vi "viewerDisplay.vi"(8 "error in (no error)":errorcluster, 9 "closeEvent":refnum<user-event>, 10 "snapperEvents":T1, 11 "Views.lvlib:Camera.lvlib:Snapper in":refnum<class "Snapper.lvclass">) -> (0 "error out":errorcluster, 3 "Views.lvlib:Camera.lvlib:Snapper out":refnum<class "Snapper.lvclass">)   [LabVIEW 2009]
uses:
  Snapper.lvclass
panel:
  out "y profile":cluster{"Pixels Line":sgl[], i32[]}(graph)
  out "X Profile":cluster{"x0":sgl, "dx":sgl, "Pixels Line":sgl[]}(graph)
  in  "Scrollbar":i32(c297)
  out "Path":path
  out "Image":T2(plugin-control)
  in  "close":bool
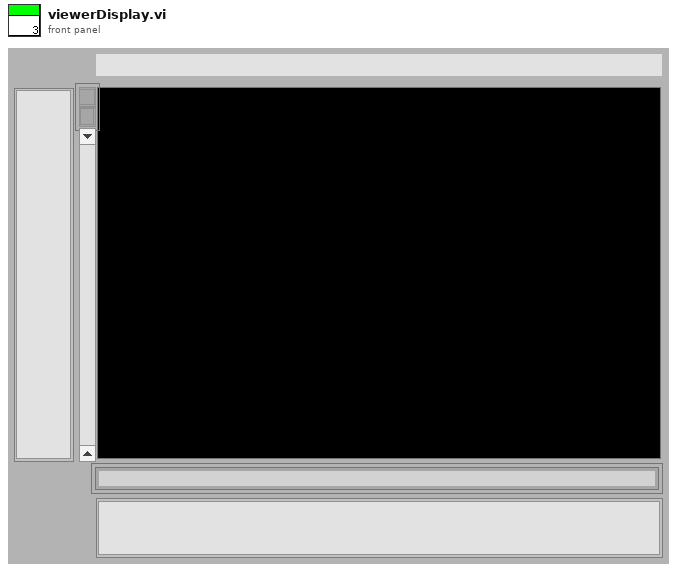
[diagram p1: front panel]
types:
  T1 = cluster{"frontEndEvents":cluster{"snapShotEvent":refnum<user-event>, "stopShooting":refnum<user-event>, "userSnapShot":refnum<user-event>}, "backEndEvents":cluster{"picture":refnum<user-event>}}
  T2 = typedef "IMAQ Image.ctl" = refnum<image>
  T3 = cluster{"snapShotEvent":refnum<user-event>, "stopShooting":refnum<user-event>, "userSnapShot":refnum<user-event>}
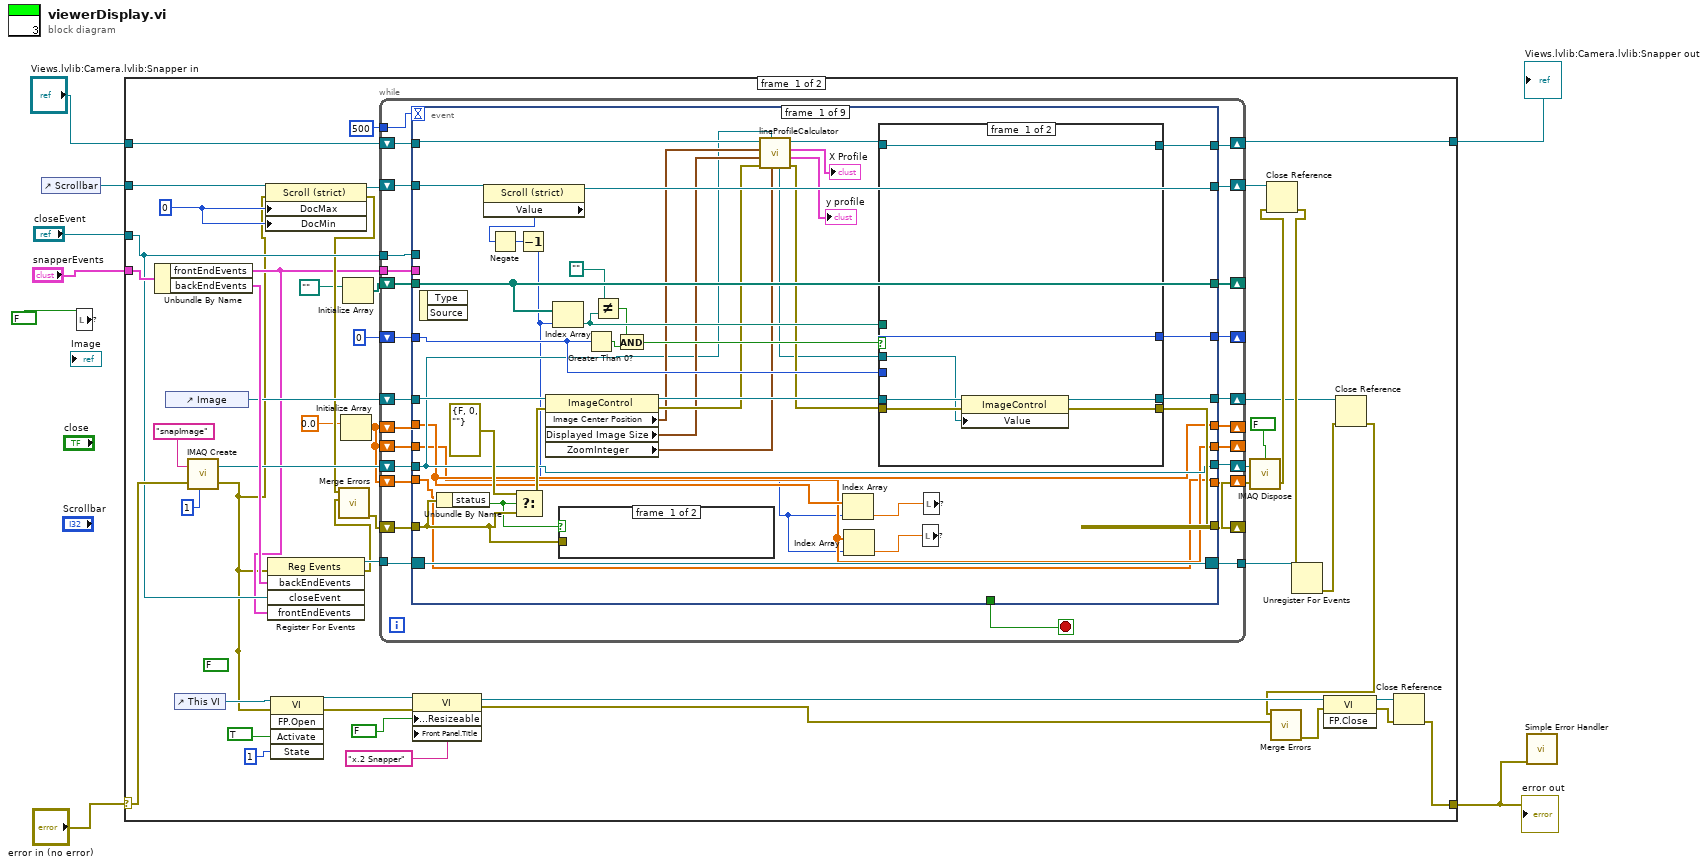
[diagram p0: block diagram]
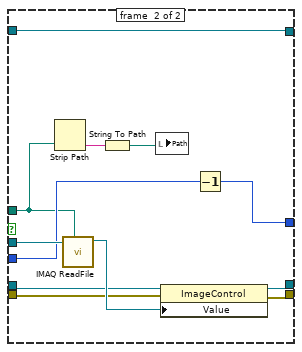
[diagram p2: hidden frame]
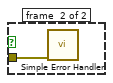
[diagram p3: hidden frame]
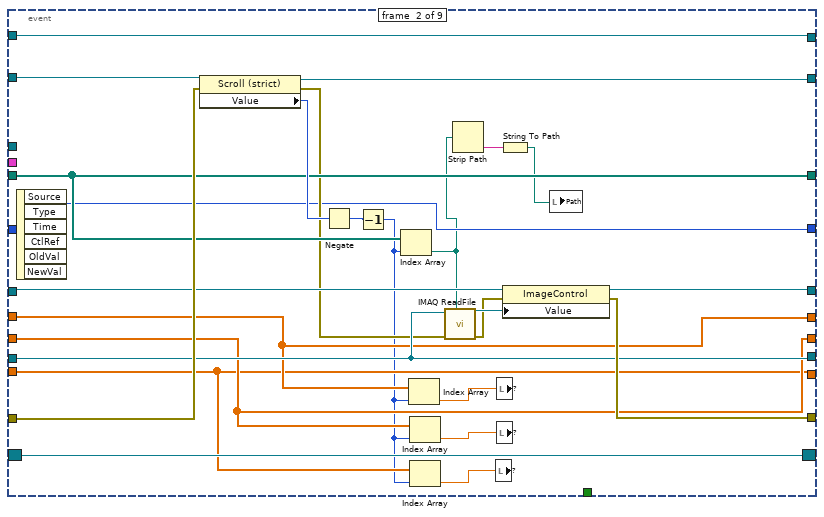
[diagram p4: hidden frame]
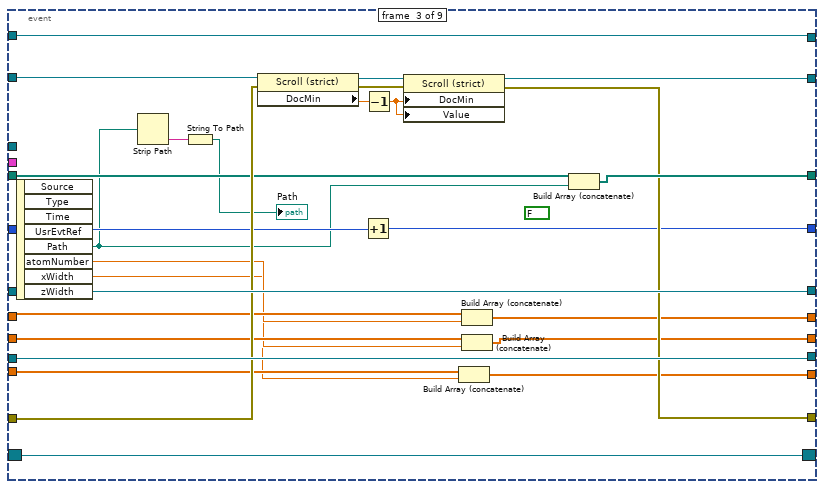
[diagram p5: hidden frame]
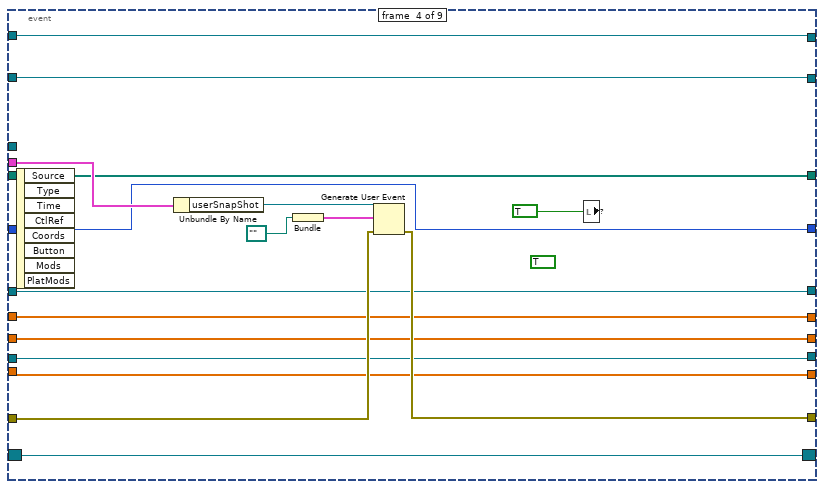
[diagram p6: hidden frame]
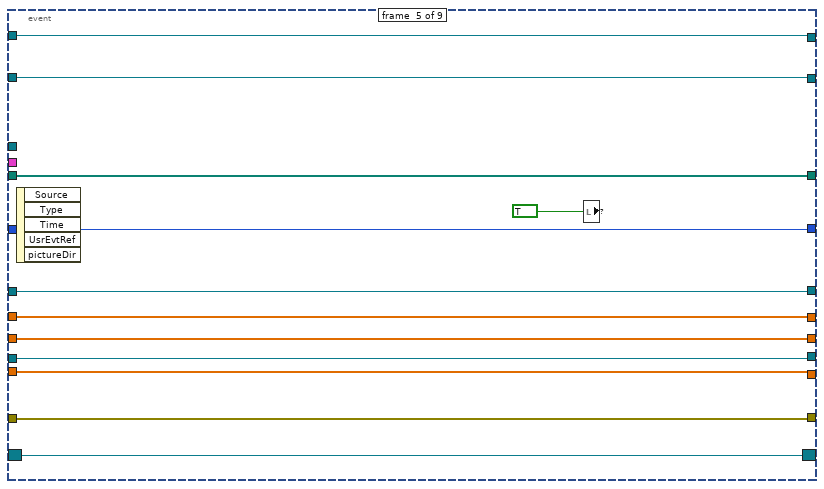
[diagram p7: hidden frame]
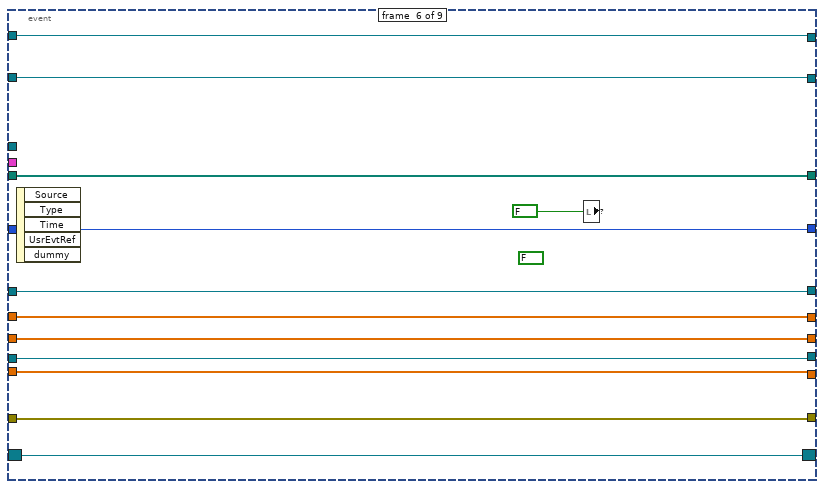
[diagram p8: hidden frame]
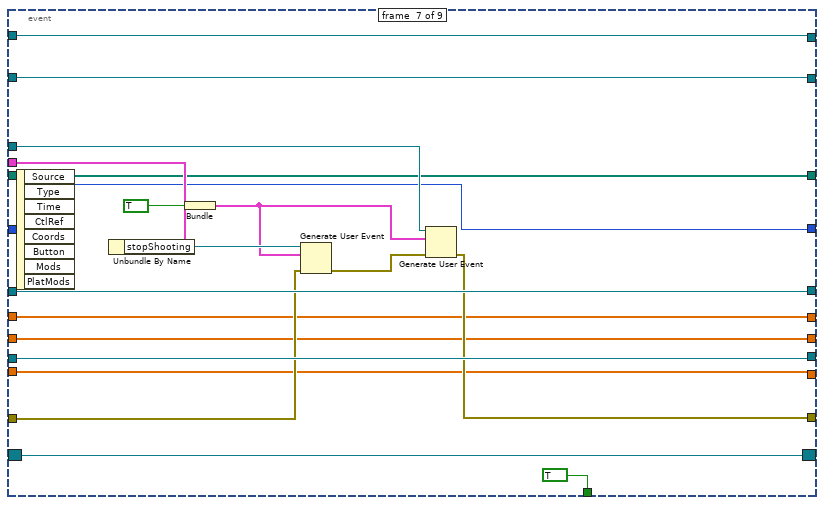
[diagram p9: hidden frame]
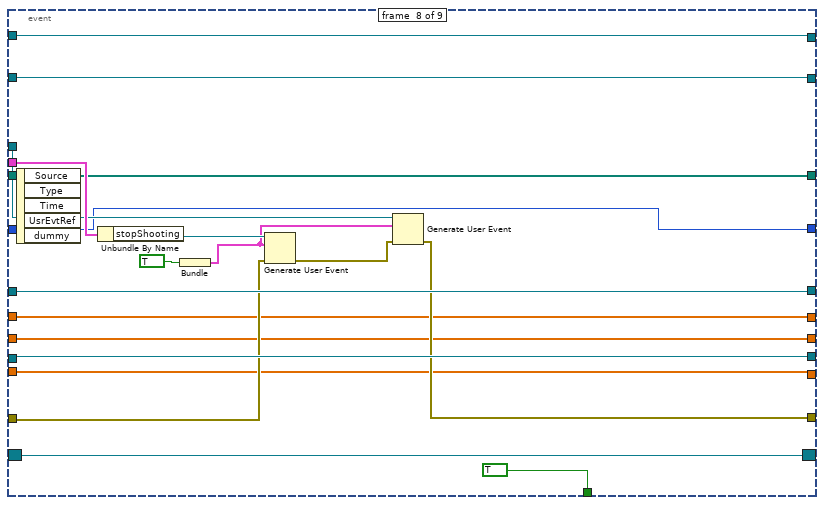
[diagram p10: hidden frame]
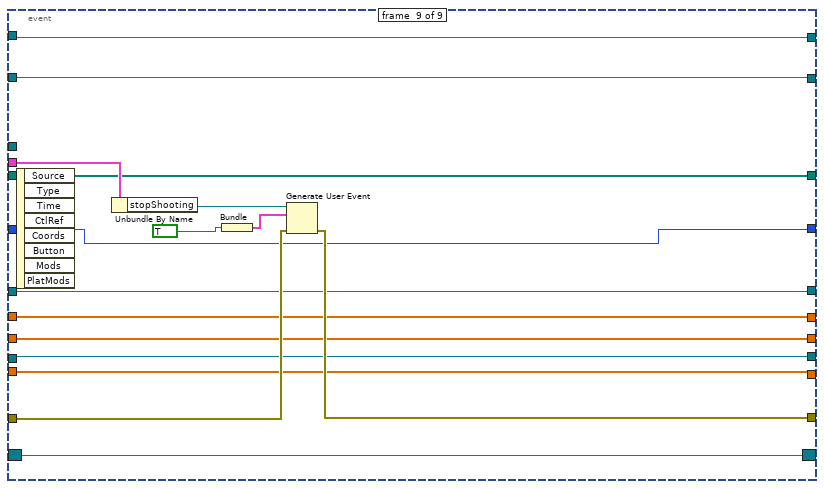
[diagram p11: hidden frame]
diagram:
  n1 = control-ref of="Scrollbar"() -> (w2:refnum<vi>)
  n2 = local write item#-1(FALSE) -> ()
  n3 = case shown="No Error" "error in (no error)" {
    selector: "error in (no error)" -> [w51 w296]
    tunnel: [w38 w296] -> w1
    tunnel: [w25 w295] -> w6
    tunnel: "Views.lvlib:Camera.lvlib:Snapper in" -> [w26 w295]
    tunnel: "snapperEvents" -> [w57 _]
    tunnel: "closeEvent" -> [w37 _]
    tunnel: w2 -> [w36 _]
    frame #0 {
      w18 = FALSE
      w34 = 0
      n4 = Unbundle By Name(w57) -> ("frontEndEvents"=w20:T3, "backEndEvents"=w55:cluster{"picture":refnum<user-event>})
      n5 = control-ref of="Image"() -> (w50:refnum<vi>)
      n6 = control-ref of="This VI"() -> (w44:refnum<vi>)
      n7 = call "IMAQ Create"("Image Name"="snapImage", "Image Type"=1, "error in (no error)"=w51) -> ("New Image"=w53:T2, "error out"=w19:errorcluster)  [unwired: 2 in]
      n8 = property class="Scroll (strict)"(reference=w36, error in=w19, "DocMax"=w34, "DocMin"=w34) -> (reference out=w35:refnum<vi>, error out=w33:errorcluster)
      n9 = register-events(error in=w19, w55, w37, w20) -> (reference out=w56:refnum<event-registration>, error out=w32:errorcluster)  [unwired: 1 in]
      n10 = invoke class="VI" method="FP.Open"(reference=w44, error in=w19, "Activate"=TRUE, "State"=1) -> (reference out=w40:refnum<vi>, error out=w39:errorcluster)  [unwired: 1 in, 3 out]
      n11 = call <vilib>:"Merge Errors.vi"("error in 2 (no error)"=w32, "error in 1 (no error)"=w33) -> ("error out"=w31:errorcluster)  [unwired: 5 in]
      n12 = Initialize Array(0.0) -> (w9:dbl[])  [unwired: 1 in]
      n13 = Initialize Array(path "") -> (w29:path[])  [unwired: 1 in]
      n14 = while {
        tunnel: w20 -> [w83]
        tunnel: w56 -> [w82]
        shift-right: [w75] -> w48
        shift-left: w53 -> [w80]
        shift-right: [w78] -> w12
        shift-left: w50 -> [w79]
        shift-right: [w77] -> w47
        shift-left: w31 -> [w81]
        tunnel: [w76] -> w46
        tunnel: w37 -> [w73]
        shift-right: [w71] -> w30
        shift-left: w35 -> [w72]
        shift-right: [w70] -> _
        shift-left: w29 -> [w69]
        tunnel: 500 -> [w68]
        shift-right: [w66] -> w25
        shift-left: w26 -> [w67]
        shift-right: [w64] -> _
        shift-left: 0 -> [w65]
        shift-right: [w61] -> _
        shift-left: w9 -> [w63]
        shift-right: [w60] -> _
        shift-left: w9 -> [w62]
        shift-right: [w58] -> _
        shift-left: w9 -> [w59]
        stop <- w74 stop-if-true
        n15 = event shown="[4] <frontEndEvents.snapShotEvent>: User Event" {
          selector: w82 -> [w122 w162 w197 w210 w227 w240 w258 w277 w288]
          dyn-events: [w122 w162 w197 w210 w227 w240 w258 w277 w288] -> w76
          timeout: w68 -> [_ _ _ _ _ _ _ _ _]
          tunnel: w83 -> [_ _ _ w215 _ _ w252 w274 w294]
          tunnel: w81 -> [w115 w166 w186 w212 w221 w233 w249 w271 w290]
          tunnel: w80 -> [w91 w158 w187 w209 w226 w239 w257 w276 w287]
          tunnel: w79 -> [w101 w165 w188 w208 w225 w238 w256 w275 w286]
          tunnel: [w91 w158 w187 w209 w226 w239 w257 w276 w287] -> w75
          tunnel: [w106 w164 w188 w208 w225 w238 w256 w275 w286] -> w78
          tunnel: [w103 w163 w183 w211 w221 w233 w254 w267 w289] -> w77
          tunnel: [_ _ _ _ _ _ TRUE TRUE _] -> w74
          tunnel: w73 -> [_ _ _ _ _ _ w255 w270 _]
          tunnel: w72 -> [w119 w168 w196 w205 w224 w236 w247 w266 w285]
          tunnel: [w116 w167 w192 w205 w224 w236 w247 w266 w285] -> w71
          tunnel: [w120 w160 w190 w204 w223 w235 w246 w265 w284] -> w70
          tunnel: w69 -> [w120 w160 w185 w204 w223 w235 w246 w265 w284]
          tunnel: w67 -> [w100 w155 w189 w203 w222 w234 w245 w264 w283]
          tunnel: [w107 w155 w189 w203 w222 w234 w245 w264 w283] -> w66
          tunnel: w65 -> [w108 w153 w182 w201 w219 w231 w244 w263 w282]
          tunnel: [w105 w153 w181 w201 w219 w231 w244 w263 w282] -> w64
          tunnel: w63 -> [w89 w152 w180 w200 w218 w230 w243 w262 w281]
          tunnel: w62 -> [w88 w151 w177 w199 w217 w229 w242 w261 w280]
          tunnel: [w89 w152 w178 w200 w218 w230 w243 w262 w281] -> w61
          tunnel: [w88 w151 w175 w199 w217 w229 w242 w261 w280] -> w60
          tunnel: w59 -> [w84 w148 w174 w198 w216 w228 w241 w260 w279]
          tunnel: [w84 w148 w172 w198 w216 w228 w241 w260 w279] -> w58
          event #0 {
            n16 = event-data() -> ()  [unwired: 1 in, 2 out]
            n17 = Unbundle By Name(w115) -> ("status"=w114:bool)
            n18 = property class="Scroll (strict)"(reference=w119) -> (reference out=w116:refnum<vi>, "Value"=w118:i32)  [unwired: 1 in, 1 out]
            n19 = Negate(x=w118) -> (-x=w117:i32)
            n20 = Select(t=errorcluster {"status"=FALSE, "code"=0, "source"=""} ("error out"), s=w114, f=w115) -> (s? t:f=w104:errorcluster)
            n21 = Decrement(x=w117) -> (x-1=w87:i32)
            n22 = property class="ImageControl"(reference=w101, error in=w104) -> (reference out=w102:refnum<vi>, error out=w95:errorcluster, "Image Center Position"=w94:cluster{"X":u32, "Y":u32}, "Displayed Image Size"=w93:cluster{"Width":u32, "Height":u32}, "ZoomInteger"=w92:cluster{"X":i32, "Y":i32})
            n23 = Index Array(array=w120, index=w87) -> (element=w112:path)
            n24 = case shown="True" w114 {
              tunnel: w115 -> [_ w142]
              frame #0 {
              }
              frame #1 {
                n25 = call <vilib>:"Simple Error Handler.vi"("error in (no error)"=w142) -> ()  [unwired: 4 in, 5 out]
              }
            }
            n26 = Greater Than 0?(x=w108) -> (x > 0?=w109:bool)
            n27 = Not Equal?(x=path "", y=w112) -> (x != y?=w110:bool)
            n28 = And(x=w110, y=w109) -> (x .and. y?=w111:bool)
            n29 = call "lineProfileCalculator.vi"("ZoomInteger"=w92, "Image"=w91, "error in (no error)"=w95, "Displayed Image Size"=w93, "Image Center Position"=w94, "Snapper in"=w100) -> ("error out"=w96:errorcluster, "y profile"=→"y profile":cluster{"Pixels Line":sgl[], i32[]}, "X Profile"=→"X Profile":cluster{"x0":sgl, "dx":sgl, "Pixels Line":sgl[]}, "Snapper out"=w99:refnum<class "Snapper.lvclass">, "Image out"=w90:T2)  [unwired: 1 in]
            n30 = Index Array(array=w89, index=w87) -> (element=w86:dbl)
            n31 = Index Array(array=w88, index=w87) -> (element=w85:dbl)
            n32 = case shown="True" w111 {
              tunnel: w90 -> [w123 w141]
              tunnel: w112 -> [_ w132]
              tunnel: w108 -> [w128 w140]
              tunnel: w102 -> [w127 w136]
              tunnel: w96 -> [w126 w135]
              tunnel: w99 -> [w129 w133]
              tunnel: [w129 w133] -> w107
              tunnel: [w125 w137] -> w106
              tunnel: [w124 w134] -> w103
              tunnel: [w128 w139] -> w105
              frame #0 {
                n33 = property class="ImageControl"(reference=w127, error in=w126, "Value"=w123) -> (reference out=w125:refnum<vi>, error out=w124:errorcluster)
              }
              frame #1 {
                n34 = Strip Path(path=w132) -> (name=w131:string)  [unwired: 1 out]
                n35 = call "IMAQ ReadFile"("File Path"=w132, "Image"=w141) -> ("Image Out"=w138:T2)  [unwired: 5 in, 4 out]
                n36 = String To Path(string=w131) -> (path=w130:path)
                n37 = local write "Path"(w130) -> ()
                n38 = property class="ImageControl"(reference=w136, error in=w135, "Value"=w138) -> (reference out=w137:refnum<vi>, error out=w134:errorcluster)
                n39 = Decrement(x=w140) -> (x-1=w139:i32)
              }
            }
            n40 = local write item#-1(w85) -> ()
            n41 = local write item#-1(w86) -> ()
          }
          event #1 {
            n42 = event-data() -> ()  [unwired: 1 in, 6 out]
            n43 = property class="Scroll (strict)"(reference=w168, error in=w166) -> (reference out=w167:refnum<vi>, error out=w157:errorcluster, "Value"=w161:i32)
            n44 = Negate(x=w161) -> (-x=w154:i32)
            n45 = Decrement(x=w154) -> (x-1=w147:i32)
            n46 = Index Array(array=w160, index=w147) -> (element=w144:path)
            n47 = Index Array(array=w152, index=w147) -> (element=w150:dbl)
            n48 = Index Array(array=w151, index=w147) -> (element=w149:dbl)
            n49 = Index Array(array=w148, index=w147) -> (element=w146:dbl)
            n50 = call "IMAQ ReadFile"("File Path"=w144, "error in (no error)"=w157, "Image"=w158) -> ("error out"=w156:errorcluster, "Image Out"=w159:T2)  [unwired: 4 in, 3 out]
            n51 = Strip Path(path=w144) -> (name=w145:string)  [unwired: 1 out]
            n52 = local write item#-1(w146) -> ()
            n53 = local write item#-1(w150) -> ()
            n54 = local write item#-1(w149) -> ()
            n55 = String To Path(string=w145) -> (path=w143:path)
            n56 = property class="ImageControl"(reference=w165, error in=w156, "Value"=w159) -> (reference out=w164:refnum<vi>, error out=w163:errorcluster)
            n57 = local write "Path"(w143) -> ()
          }
          event #2 {
            w191 = FALSE
            n58 = event-data() -> ("Path"=w169:path, "atomNumber"=w179:dbl, "xWidth"=w176:dbl, "zWidth"=w173:dbl)  [unwired: 1 in, 4 out]
            n59 = Strip Path(path=w169) -> (name=w171:string)  [unwired: 1 out]
            n60 = String To Path(string=w171) -> (path=→"Path":path)
            n61 = property class="Scroll (strict)"(reference=w196, error in=w186) -> (reference out=w195:refnum<vi>, error out=w194:errorcluster, "DocMin"=w193:dbl)
            n62 = Increment(x=w182) -> (x+1=w181:i32)
            n63 = Decrement(x=w193) -> (x-1=w184:dbl)
            n64 = property class="Scroll (strict)"(reference=w195, error in=w194, "DocMin"=w184, "Value"=w184) -> (reference out=w192:refnum<vi>, error out=w183:errorcluster)
            n65 = Build Array (concatenate)(w174, w173) -> (w172:dbl[])
            n66 = Build Array (concatenate)(w180, w179) -> (w178:dbl[])
            n67 = Build Array (concatenate)(w177, w176) -> (w175:dbl[])
            n68 = Build Array (concatenate)(w185, w169) -> (w190:path[])
          }
          event #3 {
            w202 = TRUE
            n69 = event-data() -> ()  [unwired: 1 in, 8 out]
            n70 = Unbundle By Name(w215) -> ("userSnapShot"=w214:refnum<user-event>)
            n71 = Bundle(path "") -> (w213:cluster{path})  [unwired: 1 in]
            n72 = Generate User Event(user event=w214, event data cluster=w213, error in=w212) -> (error out=w211:errorcluster)  [unwired: 1 out]
            n73 = local write item#-1(TRUE) -> ()
          }
          event #4 {
            n74 = event-data() -> ()  [unwired: 1 in, 5 out]
            n75 = local write item#-1(TRUE) -> ()
          }
          event #5 {
            w232 = FALSE
            n76 = event-data() -> ()  [unwired: 1 in, 5 out]
            n77 = local write item#-1(FALSE) -> ()
          }
          event #6 {
            n78 = event-data() -> ()  [unwired: 1 in, 8 out]
            n79 = Unbundle By Name(w252) -> ("stopShooting"=w251:refnum<user-event>)
            n80 = Bundle(TRUE) -> (w250:cluster{bool})  [unwired: 1 in]
            n81 = Generate User Event(user event=w251, event data cluster=w250, error in=w249) -> (error out=w248:errorcluster)  [unwired: 1 out]
            n82 = Generate User Event(user event=w255, event data cluster=w250, error in=w248) -> (error out=w254:errorcluster)  [unwired: 1 out]
          }
          event #7 {
            n83 = event-data() -> ()  [unwired: 1 in, 5 out]
            n84 = Unbundle By Name(w274) -> ("stopShooting"=w272:refnum<user-event>)
            n85 = Bundle(TRUE) -> (w268:cluster{bool})  [unwired: 1 in]
            n86 = Generate User Event(user event=w272, event data cluster=w268, error in=w271) -> (error out=w269:errorcluster)  [unwired: 1 out]
            n87 = Generate User Event(user event=w270, event data cluster=w268, error in=w269) -> (error out=w267:errorcluster)  [unwired: 1 out]
          }
          event #8 {
            n88 = event-data() -> ()  [unwired: 1 in, 8 out]
            n89 = Unbundle By Name(w294) -> ("stopShooting"=w293:refnum<user-event>)
            n90 = Bundle(TRUE) -> (w291:cluster{bool})  [unwired: 1 in]
            n91 = Generate User Event(user event=w293, event data cluster=w291, error in=w290) -> (error out=w289:errorcluster)  [unwired: 1 out]
          }
        }
      }
      n92 = property class="VI"(reference=w40, error in=w39, "Front Panel.Resizeable"=FALSE, "Front Panel.Title"="x.2 Snapper") -> (reference out=w17:refnum<vi>, error out=w14:errorcluster)
      n93 = call "IMAQ Dispose"("All Images? (No)"=FALSE, "Image"=w48, "error in (no error)"=w47) -> ("error out"=w24:errorcluster)  [unwired: 3 in]
      n94 = Close Reference(reference=w30, error in (no error)=w24) -> (error out=w23:errorcluster)
      n95 = Unregister For Events(event registration refnum=w46, error in=w23) -> (error out=w45:errorcluster)
      n96 = Close Reference(reference=w12, error in (no error)=w45) -> (error out=w15:errorcluster)
      n97 = call <vilib>:"Merge Errors.vi"("error in 2 (no error)"=w14, "error in 1 (no error)"=w15) -> ("error out"=w16:errorcluster)  [unwired: 5 in]
      n98 = invoke class="VI" method="FP.Close"(reference=w17, error in=w16) -> (reference out=w22:refnum<vi>, error out=w21:errorcluster)  [unwired: 1 in, 1 out]
      n99 = Close Reference(reference=w22, error in (no error)=w21) -> (error out=w38:errorcluster)
    }
    frame #1 {
    }
  }
  "error out" <- w1
  "Views.lvlib:Camera.lvlib:Snapper out" <- w6
  n100 = call <vilib>:"Simple Error Handler.vi"("error in (no error)"=w1) -> ()  [unwired: 4 in, 5 out]
